vi "detectFlyMultiImages.vi"(0 "im proc controls":T4={"Color Plane"=2, "downsampling"=24, "Filter"=enum."AutoM", "Number of Erosions"=2, "Focus threshold"=20.0, "Focus std threshold"=0.0, "background\nsubtraction"=FALSE, "Threshold"=0} {"Threshold" scale=0.0..255.0; "Color Plane" items=["Red", "Green", "Blue", "Hue", "Saturation", "Luminance", "Value", "Intensity"]}, 5 "image cluster":T3={"raw"="processed", "single channel"="processed", "focus check"="focus", "downsampled"="focus", "subtraction"="focus", "thresholded"="focus", "filtered"="focus", "cleaned"="focus", "cropped"="cropped"}, 7 "image format controls":T1={"Pixel Format"="YUV 422 Packed", "width"=2448, "height"=900, "sub image height"=600, "sub image width"=1200}) -> (4 "acquired FPS":dbl=23.880597014925375, 6 "processed FPS":dbl=23.880597014925375, 8 "Number of Particles":i32=1, 10 "Buffer Number Out":u32=414, 15 "image cluster out":T3)   [LabVIEW 2012]
uses:
  <vilib>/vision/Image Controls.llb/IMAQ Image.ctl
  GlobalBaslerCamera.vi
  <vilib>/vision/driver/NI_Vision_Acquisition_Software.lvlib
  <vilib>/vision/NI_Vision_Development_Module.lvlib
panel:
  out "Global Report":T5={"Mean Value"=1.2830653, "Standard Variation"=7.5779014, "Minimal Value"=0.0, "Maximal Value"=151.0, "Area (calibrated)"=1470000.0, "Area (pixels)"=1470000, "%"=100.0, "Calibration Valid"=TRUE} {"Mean Value" format="%.2f"; "%" format="%.2f"; "Area (calibrated)" format="%.2f"; "Maximal Value" format="%.2f"; "Minimal Value" format="%.2f"; "Standard Variation" format="%.2f"}
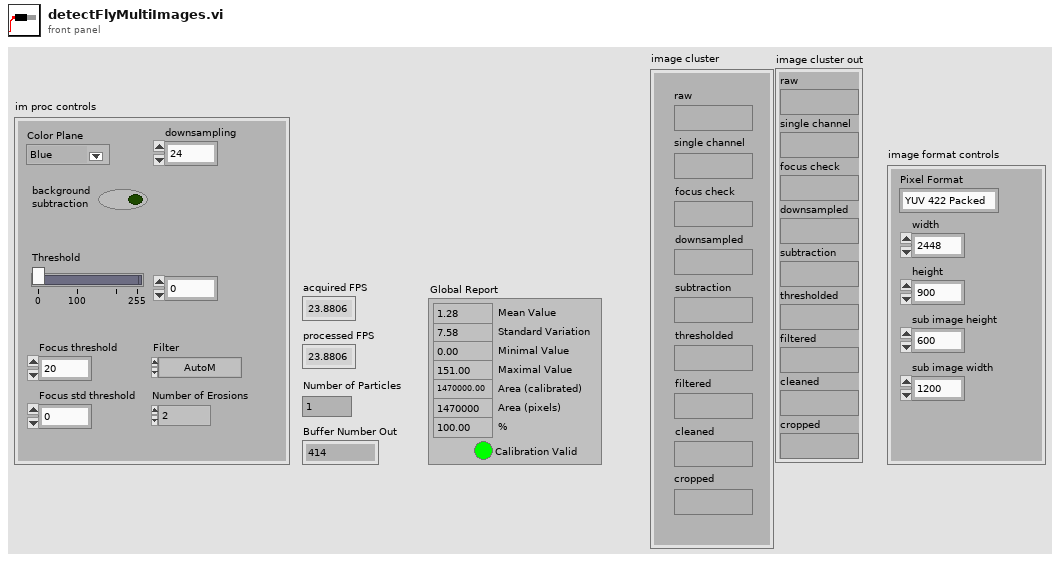
[diagram p1: front panel]
types:
  T1 = cluster{"Pixel Format":string, "width":u32, "height":u32, "sub image height":u32, "sub image width":u32}
  T2 = typedef "IMAQ Image.ctl" = refnum<image>
  T3 = cluster{"raw":T2, "single channel":T2, "focus check":T2, "downsampled":T2, "subtraction":T2, "thresholded":T2, "filtered":T2, "cleaned":T2, "cropped":T2}
  T4 = cluster{"Color Plane":i32, "downsampling":i32, "Filter":enum32{"AutoM", "Close", "Dilate", "Erode", "Gradient", "Gradient out", "Gradient in", "Hit miss", "Open", "PClose", "POpen", "Thick", "Thin"}, "Number of Erosions":i32, "Focus threshold":sgl, "Focus std threshold":sgl, "background\nsubtraction":bool, "Threshold":u8}
  T5 = cluster{"Mean Value":sgl, "Standard Variation":sgl, "Minimal Value":sgl, "Maximal Value":sgl, "Area (calibrated)":sgl, "Area (pixels)":u32, "%":sgl, "Calibration Valid":bool}
  T6 = typedef "IMAQdx.ctl" = refnum<k21>
  T7 = enum32{"Differentiation", "Gradient", "Prewitt", "Roberts", "Sigma", "Sobel"}
  T8 = enum32{"AutoM", "Close", "Dilate", "Erode", "Gradient", "Gradient out", "Gradient in", "Hit miss", "Open", "PClose", "POpen", "Thick", "Thin"}
  T9 = typedef "Particle Parameters" = i32
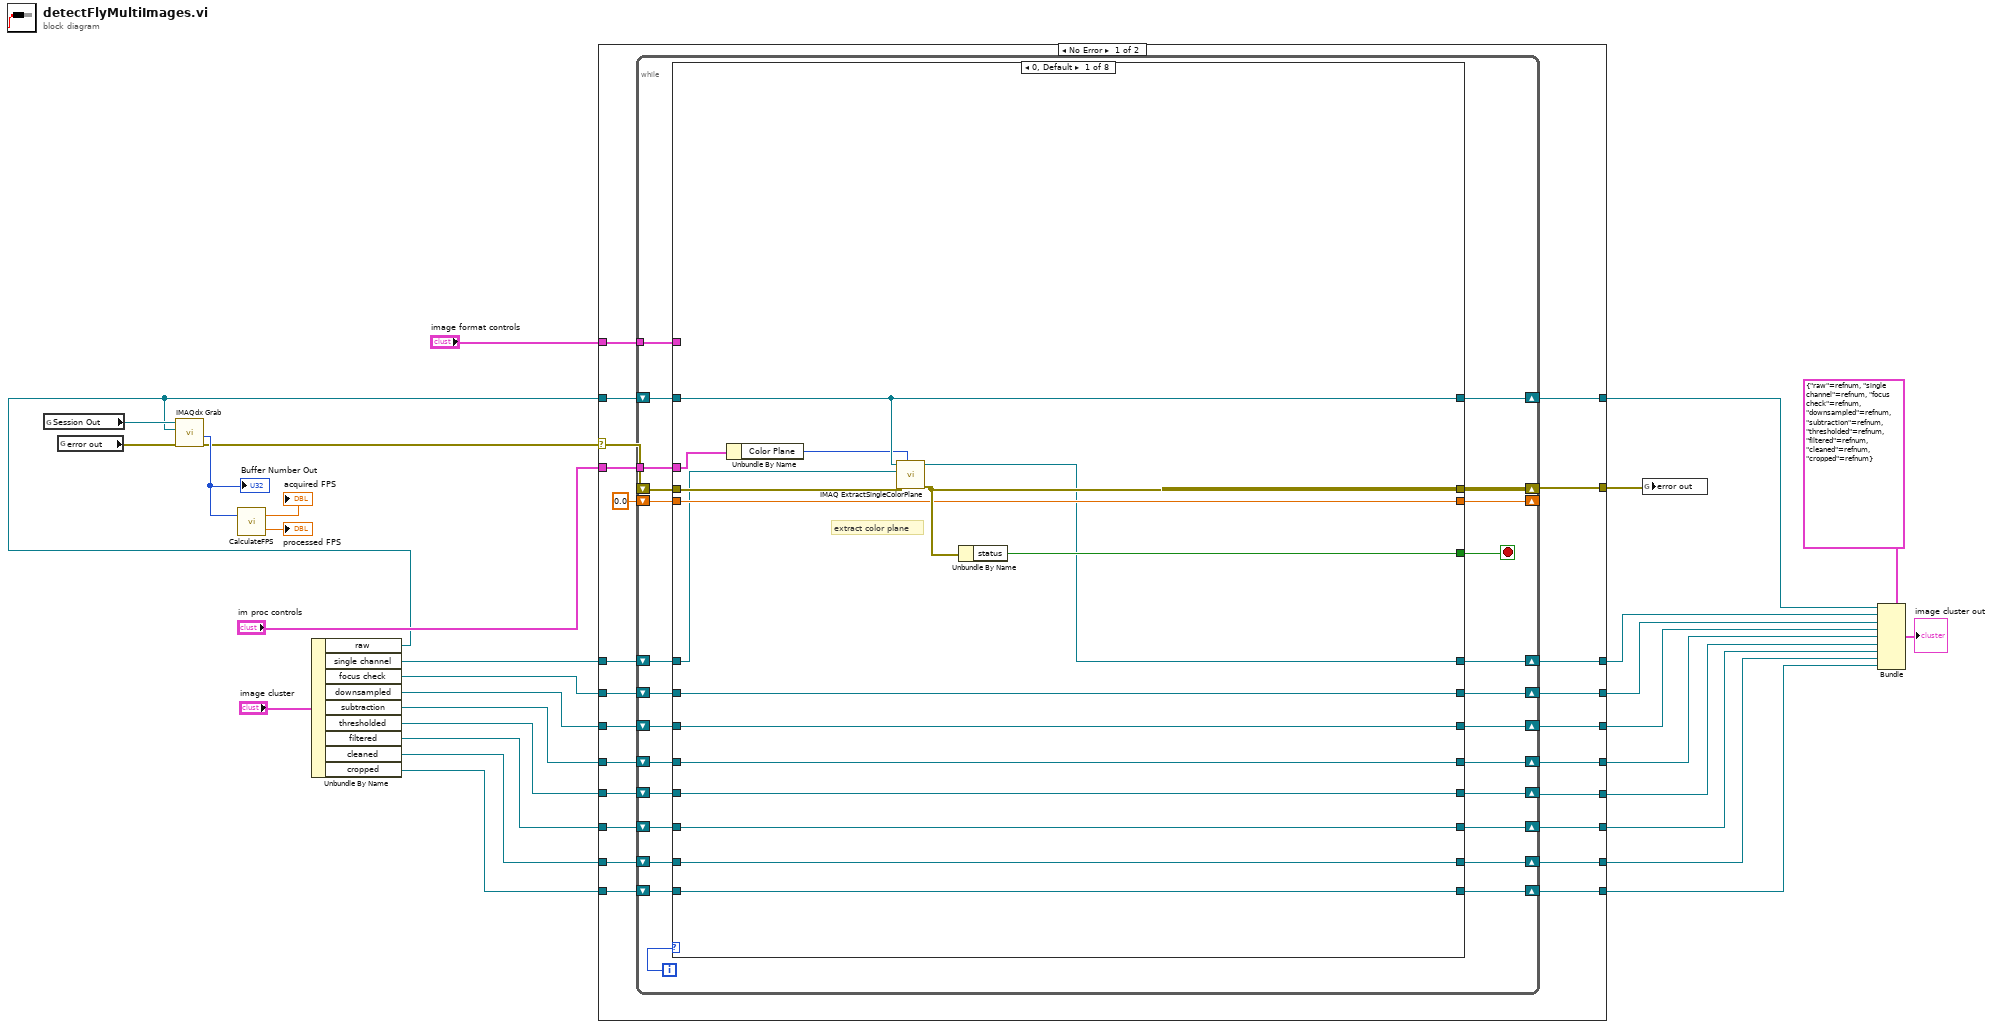
[diagram p0: block diagram]
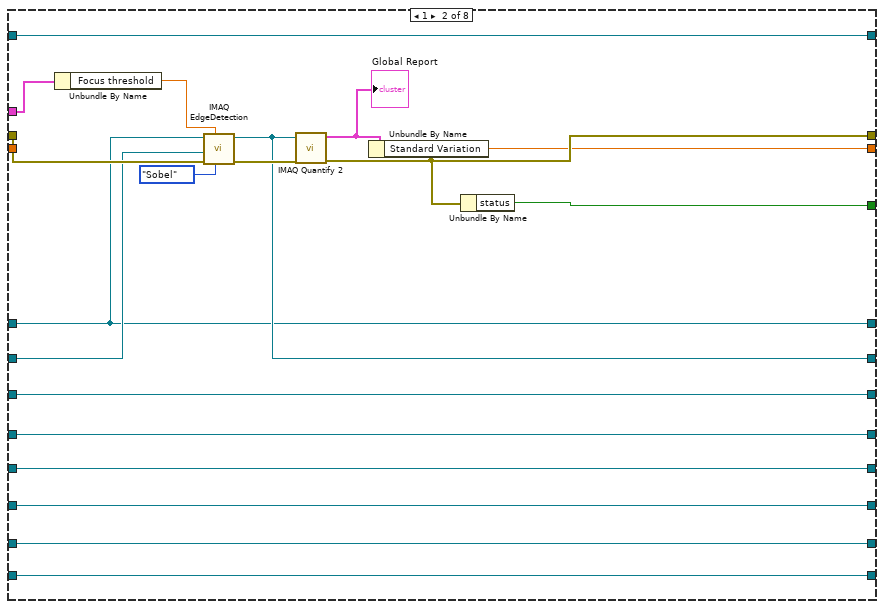
[diagram p2: hidden frame]
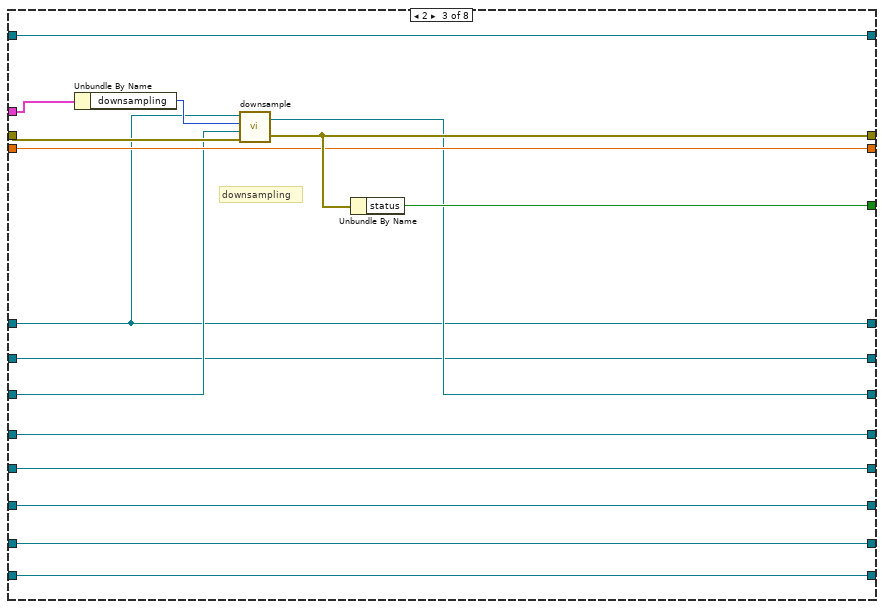
[diagram p3: hidden frame]
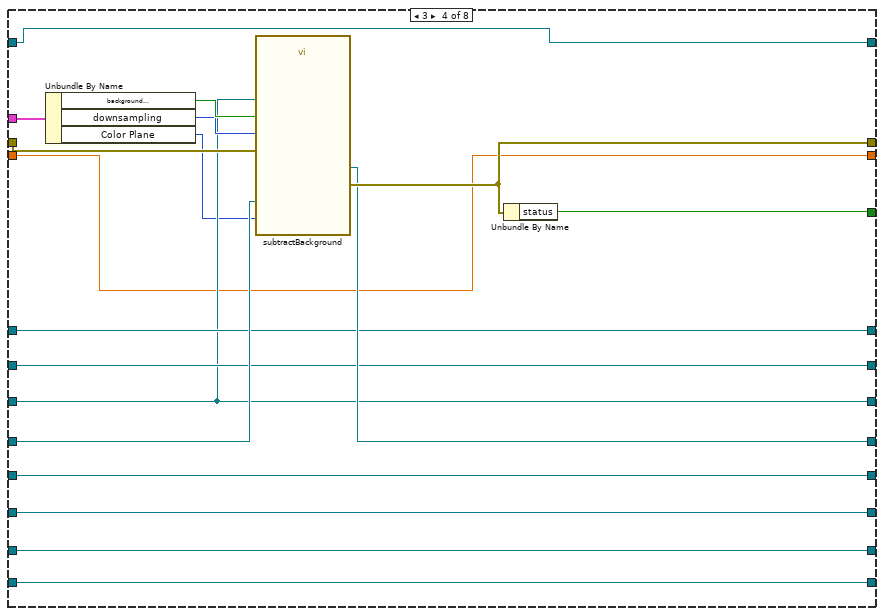
[diagram p4: hidden frame]
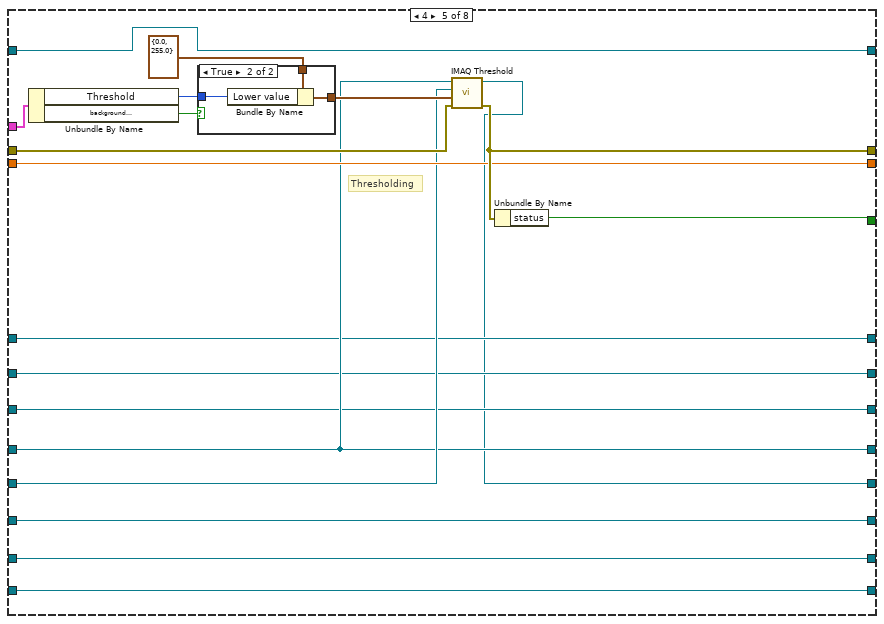
[diagram p5: hidden frame]
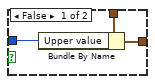
[diagram p6: hidden frame]
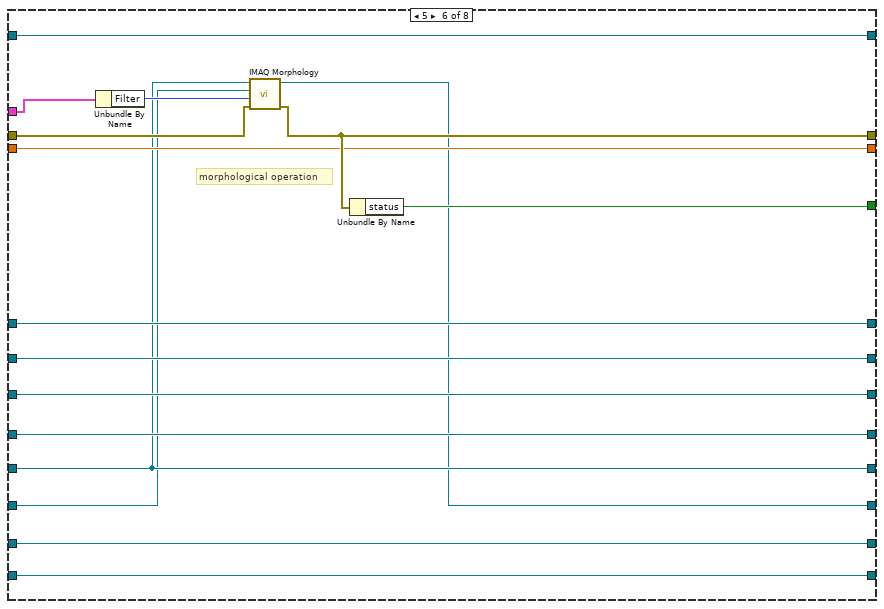
[diagram p7: hidden frame]
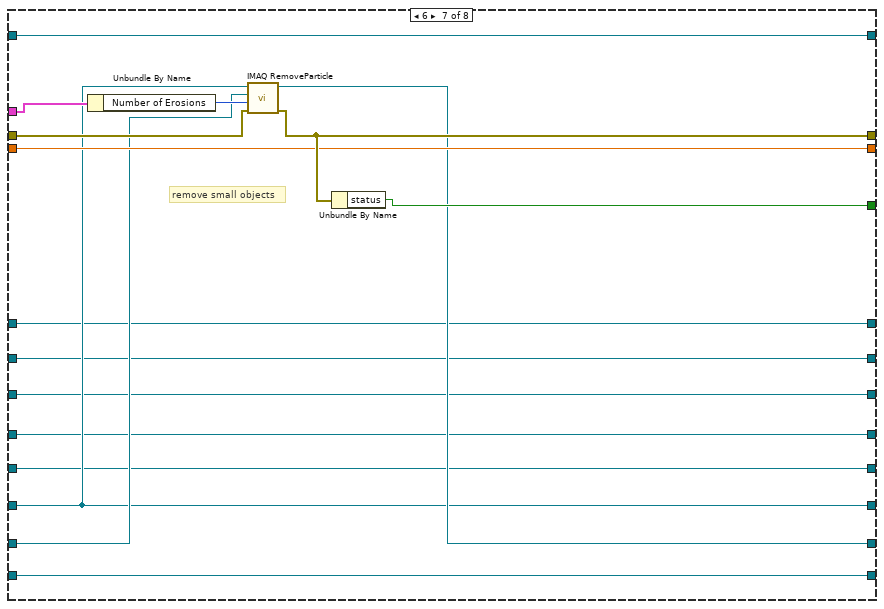
[diagram p8: hidden frame]
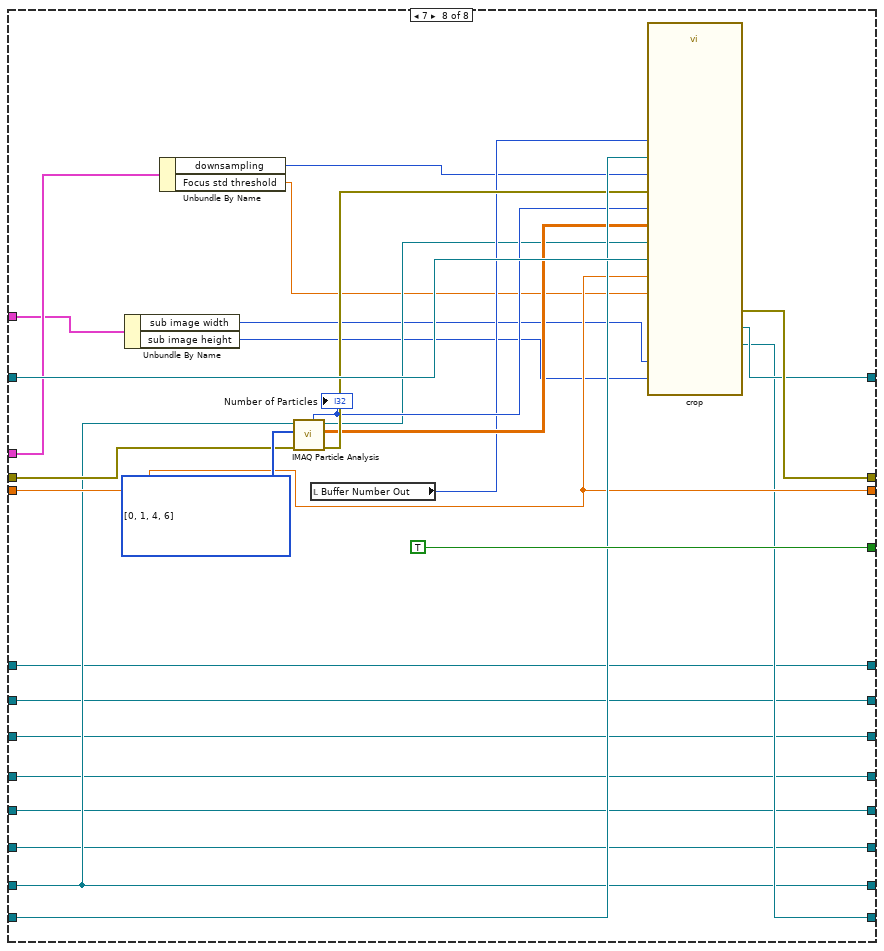
[diagram p9: hidden frame]
diagram:
  n1 = global read "GlobalBaslerCamera.vi" "Session Out"() -> (w30:T6)
  n2 = global read "GlobalBaslerCamera.vi" "error out"() -> (w29:errorcluster)
  n3 = Unbundle By Name("image cluster") -> ("raw"=w4:T2, "single channel"=w21:T2, "focus check"=w20:T2, "downsampled"=w19:T2, "subtraction"=w18:T2, "thresholded"=w17:T2, "filtered"=w16:T2, "cleaned"=w15:T2, "cropped"=w14:T2)
  n4 = call <vilib>:"IMAQdx Grab.vi"("error in"=w29, "Image In"=w4, "Session In"=w30) -> ("error out"=w26:errorcluster, "Buffer Number Out"=w28:u32)  [unwired: 1 in, 6 out]
  "Buffer Number Out" <- w28
  n5 = call "CalculateFPS.vi"("buffer number"=w28) -> ("processed FPS"=→"processed FPS":dbl, "acquired FPS"=→"acquired FPS":dbl)  [unwired: 1 in]
  n6 = case shown="No Error" w26 {
    selector: w26 -> [w53 w242]
    tunnel: w4 -> [w52 w241]
    tunnel: [w51 w242] -> w25
    tunnel: [w50 w241] -> w13
    tunnel: w14 -> [w49 w233]
    tunnel: "im proc controls" -> [w47 _]
    tunnel: w21 -> [w46 w240]
    tunnel: w20 -> [w45 w239]
    tunnel: w19 -> [w44 w238]
    tunnel: w18 -> [w43 w237]
    tunnel: w17 -> [w42 w236]
    tunnel: w16 -> [w41 w235]
    tunnel: w15 -> [w40 w234]
    tunnel: [w39 w234] -> w6
    tunnel: [w38 w235] -> w7
    tunnel: [w37 w236] -> w8
    tunnel: [w36 w237] -> w9
    tunnel: [w35 w238] -> w10
    tunnel: [w34 w239] -> w11
    tunnel: [w33 w240] -> w12
    tunnel: [w32 w233] -> w5
    tunnel: "image format controls" -> [w31 _]
    frame No Error {
      n7 = while {
        shift-right: [w78] -> w51
        shift-left: w53 -> [w76]
        shift-right: [w73] -> _
        shift-left: sgl 0.0 ("Standard Variation") -> [w72]
        tunnel: w47 -> [w71]
        shift-right: [w75] -> w50
        shift-left: w52 -> [w77]
        shift-right: [w69] -> w33
        shift-left: w46 -> [w70]
        shift-right: [w66] -> w34
        shift-left: w45 -> [w67]
        shift-right: [w64] -> w35
        shift-left: w44 -> [w65]
        shift-right: [w62] -> w36
        shift-left: w43 -> [w63]
        shift-right: [w60] -> w37
        shift-left: w42 -> [w61]
        shift-right: [w58] -> w38
        shift-left: w41 -> [w59]
        shift-right: [w56] -> w39
        shift-left: w40 -> [w57]
        shift-right: [w55] -> w32
        shift-left: w49 -> [w74]
        tunnel: w31 -> [w54]
        i -> [w79]
        stop <- w68 stop-if-true
        n8 = case shown="0, Default" w79 {
          tunnel: [w93 w110 w129 w147 w166 w188 w204 TRUE ("status")] -> w68
          tunnel: [w94 w109 w128 w143 w165 w187 w203 w226] -> w78
          tunnel: w77 -> [w92 w111 w127 w136 w158 w186 w202 w229]
          tunnel: w76 -> [w95 w108 w130 w144 w167 w189 w205 w231]
          tunnel: [w92 w111 w127 w136 w158 w186 w202 w217] -> w75
          tunnel: w74 -> [w80 w96 w115 w132 w149 w174 w190 w228]
          tunnel: [w91 w107 w126 w137 w164 w185 w201 w221] -> w73
          tunnel: w72 -> [w91 _ w126 w137 w164 w185 w201 w221]
          tunnel: w71 -> [w90 w106 w125 w148 w160 w183 w200 w219]
          tunnel: w70 -> [w88 w101 w120 w139 w153 w182 w191 w209]
          tunnel: [w87 w101 w120 w139 w153 w182 w191 w209] -> w69
          tunnel: w67 -> [w86 w104 w121 w140 w154 w181 w192 w210]
          tunnel: [w86 w103 w121 w140 w154 w181 w192 w210] -> w66
          tunnel: w65 -> [w85 w102 w123 w138 w155 w180 w193 w211]
          tunnel: [w85 w102 w122 w138 w155 w180 w193 w211] -> w64
          tunnel: w63 -> [w84 w100 w119 w142 w156 w179 w194 w212]
          tunnel: [w84 w100 w119 w141 w156 w179 w194 w212] -> w62
          tunnel: w61 -> [w83 w99 w118 w135 w157 w178 w195 w213]
          tunnel: [w83 w99 w118 w135 w152 w178 w195 w213] -> w60
          tunnel: w59 -> [w82 w98 w117 w134 w151 w177 w196 w214]
          tunnel: [w82 w98 w117 w134 w151 w176 w196 w214] -> w58
          tunnel: w57 -> [w81 w97 w116 w133 w150 w175 w198 w215]
          tunnel: [w81 w97 w116 w133 w150 w175 w197 w215] -> w56
          tunnel: [w80 w96 w115 w132 w149 w174 w190 w216] -> w55
          tunnel: w54 -> [_ _ _ _ _ _ _ w208]
          frame 0, Default {
            # "extract color plane"
            n9 = Unbundle By Name(w90) -> ("Color Plane"=w89:i32)
            n10 = call "IMAQ ExtractSingleColorPlane"("Color Plane"=w89, "error in (no error)"=w95, "Image Dst"=w88, "Image Src"=w92) -> ("error out"=w94:errorcluster, "Image Dst Out"=w87:T2)  [unwired: 6 in]
            n11 = Unbundle By Name(w94) -> ("status"=w93:bool)
          }
          frame 1 {
            n12 = Unbundle By Name(w106) -> ("Focus threshold"=w105:sgl)
            n13 = call "IMAQ EdgeDetection"("Method"=T7."Sobel", "Threshold Value"=w105, "error in (no error)"=w108, "Image Dst"=w104, "Image Src"=w101) -> ("error out"=w113:errorcluster, "Image Dst Out"=w103:T2)  [unwired: 5 in]
            n14 = call "IMAQ Quantify 2"("error in (no error)"=w113, "Image"=w103) -> ("error out"=w109:errorcluster, "Global Report"=w112:T5)  [unwired: 7 in, 1 out]
            "Global Report" <- w112
            n15 = Unbundle By Name(w112) -> ("Standard Variation"=w107:sgl)
            n16 = Unbundle By Name(w109) -> ("status"=w110:bool)
          }
          frame 2 {
            # "downsampling"
            n17 = Unbundle By Name(w125) -> ("downsampling"=w124:i32)
            n18 = call "downsample.vi"("error in"=w130, "img dst"=w123, "downsampling"=w124, "img src"=w120) -> ("error out"=w128:errorcluster, "Image Dst Out"=w122:T2)
            n19 = Unbundle By Name(w128) -> ("status"=w129:bool)
          }
          frame 3 {
            n20 = Unbundle By Name(w148) -> ("background\nsubtraction"=w146:bool, "downsampling"=w145:i32, "Color Plane"=w131:i32)
            n21 = call "subtractBackground.vi"("Color Plane"=w131, "subtraction result"=w142, "error IO"=w144, "downsampling"=w145, "saveBG"=w146, "processed image"=w138) -> ("error out"=w143:errorcluster, "processed image out"=w141:T2)  [unwired: 4 in]
            n22 = Unbundle By Name(w143) -> ("status"=w147:bool)
          }
          frame 4 {
            # "Thresholding"
            n23 = Unbundle By Name(w160) -> ("Threshold"=w163:u8, "background\nsubtraction"=w159:bool)
            n24 = case shown="True" w159 {
              tunnel: w163 -> [w170 w173]
              tunnel: [w169 w172] -> w162
              tunnel: cluster{"Lower value":sgl, "Upper value":sgl} {"Lower value"=0.0, "Upper value"=255.0} ("Range") -> [w168 w171]
              frame False {
                n25 = Bundle By Name(cluster=w168, "Upper value"=w170) -> (w169:cluster{"Lower value":sgl, "Upper value":sgl})
              }
              frame True {
                n26 = Bundle By Name(cluster=w171, "Lower value"=w173) -> (w172:cluster{"Lower value":sgl, "Upper value":sgl})
              }
            }
            n27 = call "IMAQ Threshold"("error in (no error)"=w167, "Range"=w162, "Image Dst"=w157, "Image Src"=w156) -> ("error out"=w165:errorcluster, "Image Dst Out"=w152:T2)  [unwired: 6 in]
            n28 = Unbundle By Name(w165) -> ("status"=w166:bool)
          }
          frame 5 {
            # "morphological operation"
            n29 = Unbundle By Name(w183) -> ("Filter"=w184:T8)
            n30 = call "IMAQ Morphology"("error in (no error)"=w189, "Operation"=w184, "Image Dst"=w177, "Image Src"=w178) -> ("error out"=w187:errorcluster, "Image Dst Out"=w176:T2)  [unwired: 6 in]
            n31 = Unbundle By Name(w187) -> ("status"=w188:bool)
          }
          frame 6 {
            # "remove small objects"
            n32 = Unbundle By Name(w200) -> ("Number of Erosions"=w199:i32)
            n33 = call "IMAQ RemoveParticle"("error in (no error)"=w205, "Number of Erosion"=w199, "Image Dst"=w198, "Image Src"=w196) -> ("error out"=w203:errorcluster, "Image Dst Out"=w197:T2)  [unwired: 6 in]
            n34 = Unbundle By Name(w203) -> ("status"=w204:bool)
          }
          frame 7 {
            w232 = T9[] [0, 1, 4, 6] items=["Center of Mass X", "Center of Mass Y", "First Pixel X", "First Pixel Y", "Bounding Rect Left", "Bounding Rect Top", "Bounding Rect Right", "Bounding Rect Bottom", "Max Feret Diameter Start X", "Max Feret Diameter Start Y", "Max Feret Diameter End X", "Max Feret Diameter End Y", "Max Horiz. Segment Length Left", "Max Horiz. Segment Length Right", "Max Horiz. Segment Length Row", "-", "Bounding Rect Width", "Bounding Rect Height", "Bounding Rect Diagonal", "Perimeter", "Convex Hull Perimeter", "Holes' Perimeter", "Max Feret Diameter", "Equivalent Ellipse Major Axis", "Equivalent Ellipse Minor Axis", "Equivalent Ellipse Minor Axis (Feret)", "Equivalent Rect Long Side", "Equivalent Rect Short Side", "Equivalent Rect Diagonal", "Equivalent Rect Short Side (Feret)", "Average Horiz. Segment Length", "Average Vert. Segment Length", "Hydraulic Radius", "Waddel Disk Diameter", "-", "Area", "Holes' Area", "Particle & Holes' Area", "Convex Hull Area", "Image Area", "-", "Number of Holes", "Number of Horiz. Segments", "Number of Vert. Segments", "-", "Orientation", "Max Feret Diameter Orientation", "-", "% Area/Image Area", "% Area/(Particle & Holes' Area)", "Ratio of Equivalent Ellipse Axes", "Ratio of Equivalent Rect Sides", "-", "Elongation Factor", "Compactness Factor", "Heywood Circularity Factor", "Type Factor", "-", "Sum X", "Sum Y", "Sum XX", "Sum XY", "Sum YY", "Sum XXX", "Sum XXY", "Sum XYY", "Sum YYY", "-", "Moment of Inertia XX", "Moment of Inertia XY", "Moment of Inertia YY", "Moment of Inertia XXX", "Moment of Inertia XXY", "Moment of Inertia XYY", "Moment of Inertia YYY", "Norm. Moment of Inertia XX", "Norm. Moment of Inertia XY", "Norm. Moment of Inertia YY", "Norm. Moment of Inertia XXX", "Norm. Moment of Inertia XXY", "Norm. Moment of Inertia XYY", "Norm. Moment of Inertia YYY", "Hu Moment 1", "Hu Moment 2", "Hu Moment 3", "Hu Moment 4", "Hu Moment 5", "Hu Moment 6", "Hu Moment 7"] ("Pixel Measurements")
            n35 = Unbundle By Name(w208) -> ("sub image width"=w207:u32, "sub image height"=w206:u32)
            n36 = Unbundle By Name(w219) -> ("downsampling"=w220:i32, "Focus std threshold"=w218:sgl)
            n37 = call "IMAQ Particle Analysis"("error in (no error)"=w231, "Pixel Measurements"=w232, "Image"=w215) -> ("error out"=w227:errorcluster, "Particle Measurements (Pixels)"=w225:dbl[][], "Image Out (duplicate)"=w222:T2, "Number of Particles"=w224:i32)  [unwired: 2 in, 3 out]
            "Number of Particles" <- w224
            n38 = local read "Buffer Number Out"() -> (w223:u32)
            n39 = call "crop.vi"("Particle Measurements (Pixels)"=w225, "Number of Particles"=w224, "cropWidth"=w207, "cropped Image"=w228, "std threshold"=w218, "raw image"=w229, "processed image"=w222, "downsampling"=w220, "Standard Variation"=w221, "buffer number"=w223, "cropHeight"=w206, "error in"=w227) -> ("error out"=w226:errorcluster, "raw image out"=w217:T2, "cropped image out"=w216:T2)  [unwired: 1 in]
          }
        }
      }
    }
    frame Error {
    }
  }
  n40 = global write "GlobalBaslerCamera.vi" "error out"(w25) -> ()
  n41 = Bundle(cluster=T3 {"raw"="raw", "single channel"="single channel", "focus check"="focus check", "downsampled"="downsampled", "subtraction"="subtraction", "thresholded"="thresholded", "filtered"="filtered", "cleaned"="cleaned", "cropped"="cropped"} ("image cluster out"), "raw"=w13, "single channel"=w12, "focus check"=w11, "downsampled"=w10, "subtraction"=w9, "thresholded"=w8, "filtered"=w7, "cleaned"=w6, "cropped"=w5) -> (→"image cluster out":T3)
